vi "MP_Host.vi"() -> ()   [LabVIEW 2019]
uses:
  15fe32d1-7a30-4c0c-a02d-1195f9cfa8e9.vi
  <vilib>/Analysis/baseanly.llb/Mean (DBL).vi
  <vilib>/FPGAPlugInAG/PCIe-7857/niLvFpga_Open_PCIe-7857.vi
  <vilib>/rvi/interface/common/dynamic/niFpgaDynamicAddResources.vi
  <vilib>/FPGAPlugInAG/Dynamic/niLvFpga_Reset_Dynamic.vi
  <vilib>/rvi/interface/common/niFpgaWaitOnOcc.vi
  <vilib>/Utility/error.llb/Error Cluster From Error Code.vi
  <vilib>/FPGAPlugInAG/Dynamic/niLvFpga_Run_Dynamic.vi
  <vilib>/rvi/errors/niLvFpgaAdjustHostInterfaceError.vi
  <vilib>/Utility/file.llb/Write Delimited Spreadsheet (DBL).vi
  <vilib>/FPGAPlugInAG/Dynamic/niLvFpga_Close_Dynamic.vi
  <vilib>/rvi/interface/nirviOpenFPGA/nirviOpenFPGA.xnode
  FPGA Bitfiles/mpembeexp_FPGATarget2_Mpemba1QPDcali_h0D48Adon1s.lvbitx
  Mpemba1_QPDcali.vi
  <vilib>/rvi/interface/nirviMethod/nirviMethod.xnode
  <vilib>/rvi/interface/nirviReadWriteControl/nirviReadWriteControl.xnode
  <vilib>/rvi/interface/nirviCloseFPGA/nirviCloseFPGA.xnode
  <vilib>/rvi/errors/niLvFpgaMergeErrorWithErrorCode.vi
  <vilib>/rvi/interface/Simulation/niFpgaSimulationCallBeginRW.vi
  <vilib>/Analysis/NI_AALBase.lvlib
  NiFpgaLv.dll
  <vilib>/FPGAPlugInAG/Dynamic/niLvFpga_ConfigureFifo_Dynamic.vi
  <vilib>/FPGAPlugInAG/Dynamic/niLvFpga_StartFifo_Dynamic.vi
  <vilib>/FPGAPlugInAG/Dynamic/niLvFpga_ReadFifo_Dynamic.vi
  <vilib>/FPGAPlugInAG/Dynamic/niLvFpga_StopFifo_Dynamic.vi
panel:
  in  "Flat potential\nboundary":dbl=2.0
  out "Drift":waveform(sgl)(graph)
  in  "Reset histogram":bool
  out "Initial position histogram":dynamicdata(graph)
  in  "hw cal time":sgl=50.0
  out "Elements\nremaining":dbl
  in  "AOD_AO4 2":sgl
  in  "AOD_AO0 2":sgl
  in  "Fitting Control":enum32{"Fitting Control", "Fitting Errors"}(tab)
  out "signal offset_X":sgl=5.0
  out "best fit parameters":sgl[](array[numeric])=[0.3806307, 51.013744, 11.326315, -106.03616, 2663.8608, 56396.742]
  in  "initial\nparameters":dbl[](array[numeric])=[0.0, 9.0, 9.5, 0.0, 10.0, 8.0, 0.0]
  in  "Fit?":bool
  in  "Cal px/V":dbl=64.1 format="%#_13g"
  in  "Offset":i32=5
  out "Fitting in \nprogress":bool
  out "residue":dbl
  out "error out":errorcluster
  out "smoothing error":i32
  out "Pos array":sgl[](array[numeric])
  out "Volt":sgl[](array[numeric])
  in  "Use Cal?":bool=TRUE
  in  "V_offset":sgl
  in  "Calibration":T1={"K0"=0.0, "K1"=1.0, "K2"=0.0, "K3"=0.0, "K4"=0.0, "K5"=0.0}
  in  "Bias":sgl
  in  "Fmax":sgl=50.0
  in  "cdfnorm":dbl=1.0 format="%#_16g"
  out "num of protocols":sgl=2126.0
  in  "Calibration ON/OFF":bool=TRUE
  in  "Xoffset":sgl
  in  "Yoffset":sgl
  in  "sum_offset":sgl
  out "Xpot":sgl=-0.1267538 format="%.2f"
  in  "wait time":u8=80
  in  "Temp":i8(ring)=1 items=["Cold", "Warm", "Hot"]
  in  "?":u16(ring) items=["Flat calibration", "Flat cal w drift corr", "No FB", "FB"]
  in  "DW":cluster{"xm":sgl, "Eb":sgl, "Tau":sgl, "dE":sgl}={"xm"=0.5, "Eb"=2.0, "Tau"=70.0, "dE"=1.0} {"dE" format="%#_3g"}
  in  "DL_Y":dbl=2.5 format="%#_13g"
  in  "TL_Y":dbl=2.5 format="%#_13g"
  in  "Stop":bool
  in  "FB time":u32=10
  in  "Triangle wave":T2={"signal offset_X"=5.0, "Scale X"=0.0, "signal offset_Y"=5.0, "Scale Y"=0.0, "Phase Shift"=30}
  in  "Elements":u32=100000
  in  "Data length":dbl=300.0
  out "Done saving":bool
  out "?":dbl=-19.0
  in  "Save Data":bool
  in  "mobX(px/V)":sgl=1.0
  in  "1/Xcali":sgl=1.0
  in  "DX":sgl=53.664
  out "Feedback Loop time":sgl=10.0 format="%.2f"
  out "Underflow":bool
  out "Fx out/Xcorr":sgl=5.0
  out "X":waveform(dbl)(graph)={"t0"=timestamp(0 s since 1904-01-01), "dt"=9.999999747378752e-06, "Y"=array[100000 elements]}
  out "Y":waveform(dbl)(graph)={"t0"=timestamp(0 s since 1904-01-01), "dt"=9.999999747378752e-06, "Y"=array[100000 elements]}
  out "Sum":waveform(dbl)(graph)={"t0"=timestamp(0 s since 1904-01-01), "dt"=9.999999747378752e-06, "Y"=array[100000 elements]}
  in  "Reaverage PS":bool
  out "meanX":dbl=0.10684734082818341 format="%0.5f"
  in  "Xmean":sgl
  out "PSX":dynamicdata(graph)=[{"t0"=timestamp(0 s since 1904-01-01), "dt"=1.0000000252621255, "Y"=array[50000 elements], "attributes"=variant("NI_ChannelName"=variant(string "PSD"))}]
  out "PSY":dynamicdata(graph)=[{"t0"=timestamp(0 s since 1904-01-01), "dt"=1.0000000252621255, "Y"=array[50000 elements], "attributes"=variant("NI_ChannelName"=variant(string "PSD"))}]
  out "PSsum":dynamicdata(graph)=[{"t0"=timestamp(0 s since 1904-01-01), "dt"=1.0000000252621255, "Y"=array[50000 elements], "attributes"=variant("NI_ChannelName"=variant(string "PSD"))}]
  out "Saveloop":u32
  in  "Feedback parameters":T3={"SP_QPDX"=0.0, "alpha"=0.03, "ktrap"=49.2899, "alphacounterX"=0.026}
  in  "TW freq":dbl=1.0
  in  "Normalize signal":bool=TRUE
  out "meanY":dbl=0.08517331748366355 format="%0.5f"
  out "meanZ":dbl=0.8066337188720704 format="%0.4f"
  out "?":errorcluster
  in  "file path (dialog if empty)":path=path "D:/Siddharth/Data/Mpemba replication/2025_04_28/t.txt"
  # "Set both of these to 1"
  # "Set alpha=0.1"
  # "Set cal px/V=60"
  # "Tau=protocol length in us"
  # "Total protocol length = tau+wait time"
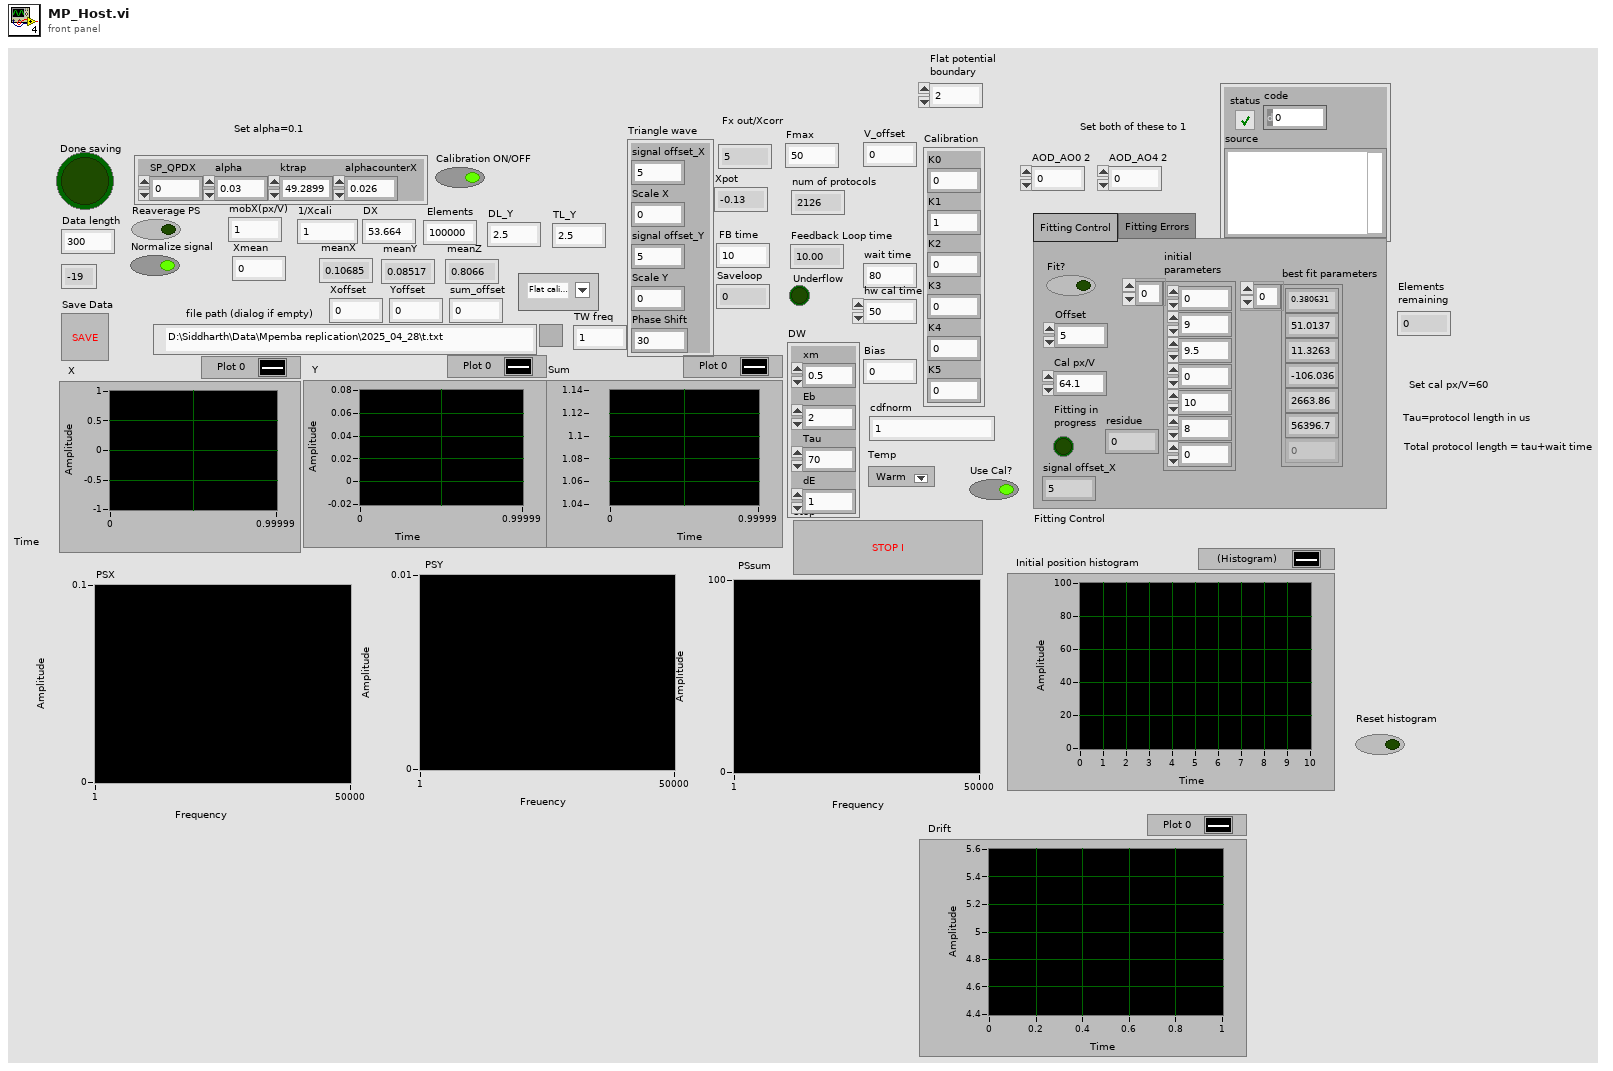
[diagram p1: front panel]
types:
  T1 = cluster{"K0":sgl, "K1":sgl, "K2":sgl, "K3":sgl, "K4":sgl, "K5":sgl}
  T2 = cluster{"signal offset_X":sgl, "Scale X":sgl, "signal offset_Y":sgl, "Scale Y":sgl, "Phase Shift":u32}
  T3 = cluster{"SP_QPDX":sgl, "alpha":sgl, "ktrap":sgl, "alphacounterX":sgl}
  T4 = cluster{"signal offset_X":sgl, dbl, "signal offset_Y":sgl, "Scale Y":sgl, u32}
  T5 = cluster{"[0]":sgl, "[1]":sgl, "[2]":sgl, "[3]":sgl, "[4]":sgl, "[5]":sgl}
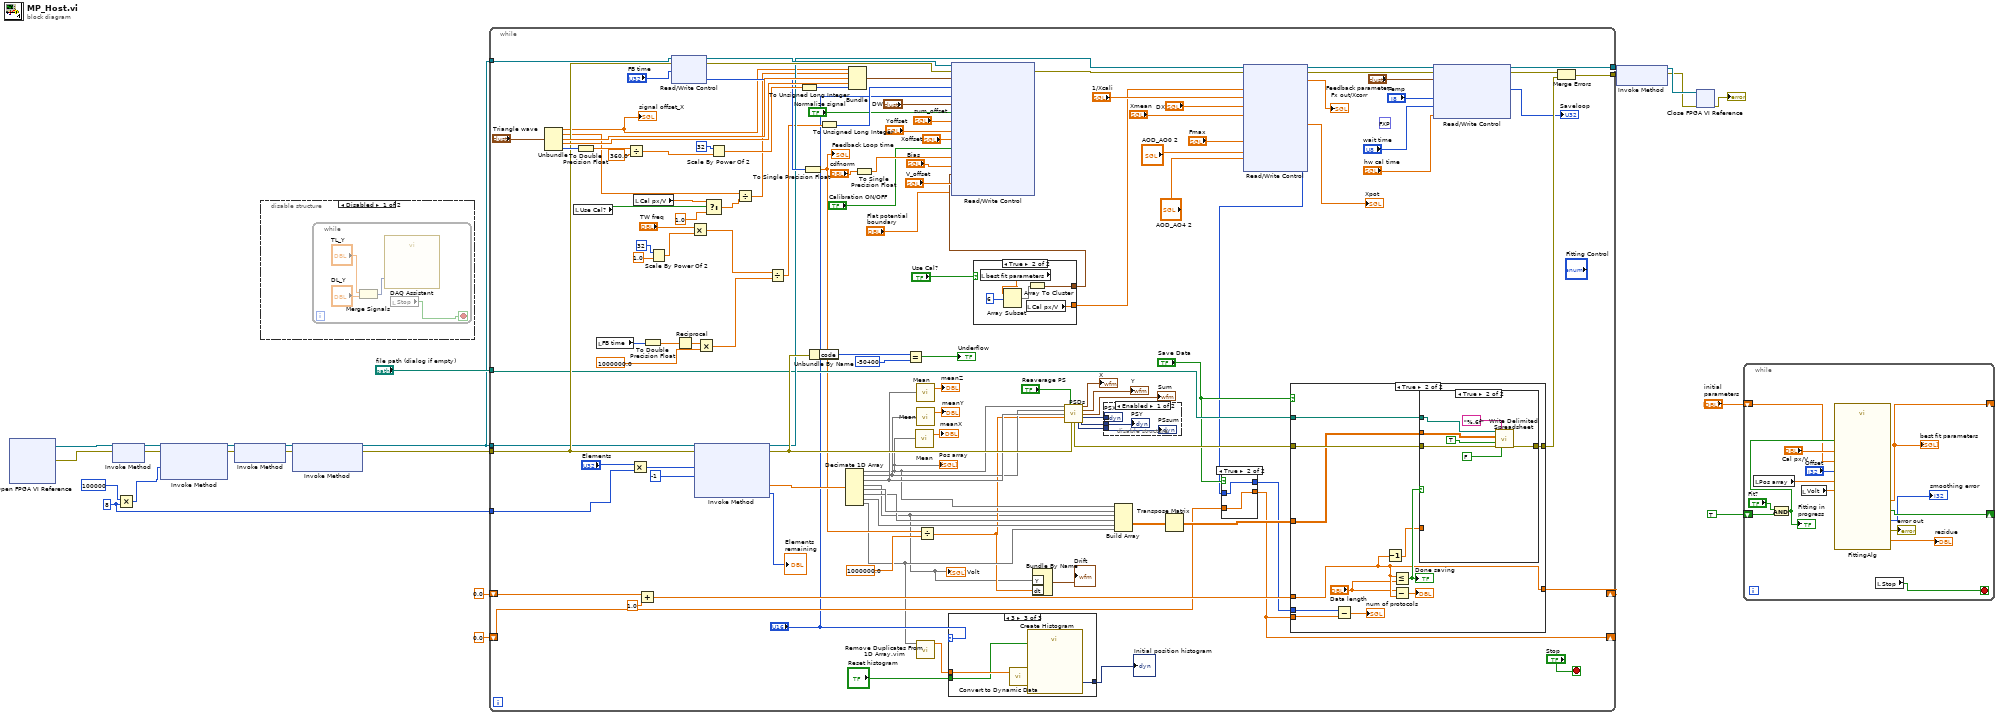
[diagram p0: block diagram]
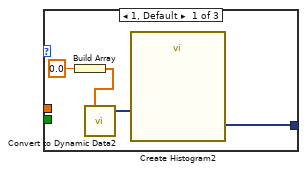
[diagram p3: hidden frame]
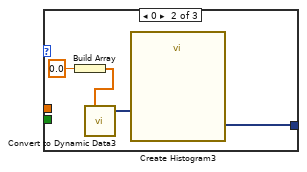
[diagram p4: hidden frame]
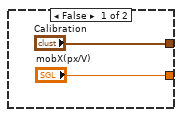
[diagram p5: hidden frame]
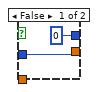
[diagram p6: hidden frame]
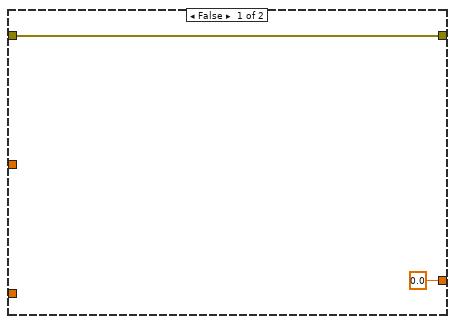
[diagram p8: hidden frame]
diagram:
  w1 = u32 8 ("y")
  n1 = xnode "Open FPGA VI Reference"() -> ("FPGA VI Reference Out"=w7:refnum<k20>, "error out"=w4:errorcluster)  [unwired: 2 in]
  n2 = xnode "Invoke Method"("FPGA VI Reference In"=w7, "error in"=w4) -> ("FPGA VI Reference Out"=w14:refnum<k20>, "error out"=w13:errorcluster)
  n3 = Multiply(x=u32 100000 ("Requested Depth"), y=w1) -> (x*y=w2:u32)
  n4 = xnode "Invoke Method"("FPGA VI Reference In"=w14, "error in"=w13, "Requested Depth"=w2) -> ("FPGA VI Reference Out"=w18:refnum<k20>, "error out"=w17:errorcluster)  [unwired: 1 out]
  n5 = xnode "Invoke Method"("FPGA VI Reference In"=w18, "error in"=w17) -> ("FPGA VI Reference Out"=w20:refnum<k20>, "error out"=w19:errorcluster)
  n6 = disable-structure shown="Disabled" {
    frame Disabled {
      n7 = while {
        stop <- w24 stop-if-true
        n8 = Merge Signals("TL_Y", "DL_Y") -> (w27:dynamicdata)
        n9 = call "DAQ Assistant"("data"=w27) -> ()  [unwired: 17 in, 2 out]
        n10 = local read "Stop"() -> (w24:bool)
      }
    }
    frame Enabled {
    }
  }
  n11 = xnode "Invoke Method"("FPGA VI Reference In"=w20, "error in"=w19) -> ("FPGA VI Reference Out"=w16:refnum<k20>, "error out"=w15:errorcluster)  [unwired: 1 in]
  n12 = while {
    tunnel: w16 -> [w127]
    tunnel: w15 -> [w128]
    tunnel: "file path (dialog if empty)" -> [w96]
    tunnel: [w120] -> w22
    tunnel: [w133] -> w21
    tunnel: w16 -> [w115]
    shift-right: [w124] -> _
    shift-left: 0.0 -> [w123]
    shift-right: [w65] -> _
    shift-left: sgl 0.0 ("num of cycles") -> [w67]
    tunnel: w1 -> [w45]
    stop <- "Stop" stop-if-true
    (unwired) fxp<+,8,7> 50.0 ("Fmax")
    n13 = Unbundle("Triangle wave") -> ("signal offset_X"=w55:sgl, "Scale X"=w33:sgl, "signal offset_Y"=w136:sgl, "Scale Y"=w135:sgl, "Phase Shift"=w137:u32)
    "signal offset_X" <- w55
    n14 = local read "Use Cal?"() -> (w31:bool)
    n15 = To Double Precision Float(number=w137) -> (double precision float=w143:dbl)
    n16 = local read "FB time"() -> (w86:u32)
    n17 = Divide(x=w143, y=360.0) -> (x/y=w141:dbl)
    n18 = Multiply(x="Elements", y=w45) -> (x*y=w129:u32)
    n19 = local read "Cal px/V"() -> (w30:dbl)
    n20 = Add(x=w123, y=1.0) -> (x+y=w125:dbl)
    n21 = To Double Precision Float(number=w86) -> (double precision float=w87:dbl)
    n22 = Scale By Power Of 2(n=i16 32, x=1.0) -> (x*2^n=w91:dbl)
    n23 = xnode "Read/Write Control"("FPGA VI Reference In"=w127, "error in"=w128, "FB Time"="FB time") -> ("FPGA VI Reference Out"=w147:refnum<k20>, "error out"=w116:errorcluster, "FB Time"=w114:u8)
    n24 = Reciprocal(x=w87) -> (1/x=w88:dbl)
    n25 = Multiply(x="TW freq", y=w91) -> (x*y=w84:dbl)
    n26 = xnode "Invoke Method"("FPGA VI Reference In"=w115, "error in"=w128, "Number of Elements"=w129, "Timeout (ms)"=-1) -> ("FPGA VI Reference Out"=w98:refnum<k20>, "error out"=w112:errorcluster, "Data"=w107:sgl[], "Elements Remaining"=→"Elements\nremaining":u32)
    n27 = Multiply(x=w88, y=1000000.0) -> (x*y=w83:dbl)
    n28 = Select(t=w30, s=w31, f=1.0) -> (s? t:f=w29:dbl)
    n29 = Scale By Power Of 2(n=i16 32, x=w141) -> (x*2^n=w139:dbl)
    n30 = Divide(x=w33, y=w29) -> (x/y=w28:dbl)
    n31 = Divide(x=w84, y=w83) -> (x/y=w82:dbl)
    n32 = To Unsigned Long Integer(number=w139) -> (unsigned 32bit integer=w134:u32)
    n33 = To Single Precision Float(number=w114) -> (single precision float=w93:sgl)
    "Feedback Loop time" <- w93
    n34 = Unbundle By Name(w112) -> ("code"=w132:i32)
    n35 = To Unsigned Long Integer(number=w82) -> (unsigned 32bit integer=w81:u32)
    n36 = Decimate 1D Array(w107) -> (w54:sgl[], w72:sgl[], w75:sgl[], w36:sgl[], w76:sgl[], w49:sgl[], w46:sgl[], w42:sgl[])
    "Pos array" <- w54
    "Volt" <- w36
    n37 = Bundle("signal offset_X"=w55, w28, "signal offset_Y"=w136, "Scale Y"=w135, w134) -> (w94:T4)  [unwired: 1 in]
    n38 = To Single Precision Float(number="cdfnorm") -> (single precision float=w59:sgl)
    n39 = Equal?(x=w132, y=-50400) -> (x = y?=→"Underflow":bool)
    n40 = call-poly <vilib>:"Mean.vi"("X"=w54) -> ("mean"=→"meanX":dbl)  [unwired: 1 out]
    n41 = call-poly <vilib>:"Mean.vi"("X"=w75) -> ("mean"=→"meanZ":dbl)  [unwired: 1 out]
    n42 = call "Remove Duplicates From 1D Array.vim"("array"=w42) -> ("array with duplicates removed"=w40:sgl[])  [unwired: 10 in]
    n43 = call-poly <vilib>:"Mean.vi"("X"=w72) -> ("mean"=→"meanY":dbl)  [unwired: 1 out]
    n44 = Divide(x=w93, y=sgl 1000000.0) -> (x/y=w37:sgl)
    n45 = case shown="3" "?" {
      tunnel: [w152 w156 w161] -> w41
      tunnel: w40 -> [_ _ w159]
      tunnel: "Reset histogram" -> [_ _ w158]
      frame 1, Default {
        n46 = Build Array(0.0 ("element")) -> (w150:dbl[])
        n47 = call "Convert to Dynamic Data2"("Array"=w150) -> ("Dynamic Data Type"=w153:dynamicdata)  [unwired: 3 in]
        n48 = call "Create Histogram2"("Signal"=w153) -> ("Histogram"=w152:dynamicdata)  [unwired: 9 in, 1 out]
      }
      frame 0 {
        n49 = Build Array(0.0 ("element")) -> (w154:dbl[])
        n50 = call "Convert to Dynamic Data3"("Array"=w154) -> ("Dynamic Data Type"=w157:dynamicdata)  [unwired: 3 in]
        n51 = call "Create Histogram3"("Signal"=w157) -> ("Histogram"=w156:dynamicdata)  [unwired: 9 in, 1 out]
      }
      frame 3 {
        n52 = call "Convert to Dynamic Data"("Array"=w159) -> ("Dynamic Data Type"=w160:dynamicdata)  [unwired: 3 in]
        n53 = call "Create Histogram"("Reset"=w158, "Signal"=w160) -> ("Histogram"=w161:dynamicdata)  [unwired: 8 in, 1 out]
      }
    }
    "Initial position histogram" <- w41
    n54 = case shown="True" "Use Cal?" {
      tunnel: ["Calibration" w168] -> w58
      tunnel: ["mobX(px/V)" w164] -> w57
      frame False {
      }
      frame True {
        n55 = local read "best fit parameters"() -> (w166:sgl[])
        n56 = Array Subset(array=w166, length=6) -> (w165:sgl[])  [unwired: 1 in]
        n57 = local read "Cal px/V"() -> (w164:dbl)
        n58 = Array To Cluster(array=w165) -> (cluster=w168:T5)
      }
    }
    n59 = xnode "Read/Write Control"("FPGA VI Reference In"=w147, "error in"=w116, "Triangle wave"=w94, "Frequency"=w81, "Enum"="?", "DW"="DW", "Normalize signal"="Normalize signal", "sum_offset"="sum_offset", "Yoffset"="Yoffset", "Xoffset"="Xoffset", "Calibration ON/OFF"="Calibration ON/OFF", "cdfnorm"=w59, "Bias"="Bias", "Calibration"=w58, "V_offset"="V_offset", "Flat potential boundary"="Flat potential\nboundary") -> ("error out"=w97:errorcluster)  [unwired: 1 out]
    n60 = Bundle By Name("Y"=w36, "dt"=w37) -> (→"Drift":waveform(sgl))  [unwired: 1 in]
    n61 = call "PSDs.vi"("X"=w54, "averaging done"="Reaverage PS", "Y"=w72, "sum"=w75, "dt"=w37, "error in (no error)"=w112) -> ("X"=→"X":waveform(dbl), "Y"=→"Y":waveform(dbl), "Sum"=→"Sum":waveform(dbl), "PSDX"=w103:dynamicdata, "error out"=w111:errorcluster, "PSDsum"=w101:dynamicdata, "PSDY"=w102:dynamicdata)  [unwired: 3 in]
    n62 = disable-structure shown="Enabled" {
      disable-tunnel: w103 -> [w175 _]
      disable-tunnel: w102 -> [w174 _]
      disable-tunnel: w101 -> [w173 _]
      frame Enabled {
        "PSX" <- w175
        "PSY" <- w174
        "PSsum" <- w173
      }
      frame Disabled {
      }
    }
    n63 = Build Array(w54, w76, w36, w49, w46, w42) -> (w118:sgl[][])
    n64 = Transpose Matrix(1:w118) -> (0:w146:dbl[][])
    n65 = xnode "Read/Write Control"("FPGA VI Reference In"=w98, "error in"=w97, "MobX(px/V)"=w57, "1/Xcali"="1/Xcali", "DX"="DX", "Xmean"="Xmean", "Fmax"="Fmax", "AOD_AO0 2"="AOD_AO0 2", "AOD_AO4 2"="AOD_AO4 2") -> ("FPGA VI Reference Out"=w122:refnum<k20>, "error out"=w121:errorcluster, "Fx out/Xcorr"=→"Fx out/Xcorr":sgl, "Xpot"=→"Xpot":sgl, "Protocol number"=w47:u32)  [unwired: 1 in]
    n66 = case shown="True" "Save Data" {
      tunnel: [w169 w171] -> w65
      tunnel: w67 -> [_ w171]
      tunnel: [i16 0 ("num of cycles") w172] -> w66
      tunnel: w47 -> [w169 w172]
      frame False {
      }
      frame True {
      }
    }
    n67 = case shown="True" "Save Data" {
      tunnel: w146 -> [_ w184]
      tunnel: w96 -> [_ w189]
      tunnel: w111 -> [w177 w188]
      tunnel: [w177 w187] -> w145
      tunnel: w125 -> [_ w183]
      tunnel: [0.0 w183] -> w124
      tunnel: w66 -> [_ w180]
      tunnel: w65 -> [_ w179]
      frame False {
      }
      frame True {
        n68 = Subtract(x=w180, y=w179) -> (x-y=→"num of protocols":sgl)
        n69 = Decrement(x=w183) -> (x-1=w182:dbl)
        n70 = Less Or Equal?(x=w183, y="Data length") -> (x <= y?=w186:bool)
        "Done saving" <- w186
        n71 = Subtract(x="Data length", y=w183) -> (x-y=→"?":dbl)
        n72 = case shown="True" w186 {
          tunnel: w184 -> [_ w191]
          tunnel: w189 -> [_ w192]
          tunnel: w188 -> [w190 w195]
          tunnel: [w190 w194] -> w187
          tunnel: w182 -> [_ _]
          frame False {
          }
          frame True {
            n73 = call-poly <vilib>:"Write Delimited Spreadsheet.vi"("file path (dialog if empty)"=w192, "format (%.3f)"="%.6f", "2D data"=w191, "append to file? (new file:F)"=TRUE, "error in (no error)"=w195, "transpose? (no:F)"=FALSE) -> ("error out"=w194:errorcluster)  [unwired: 8 in, 1 out]
          }
        }
      }
    }
    n74 = xnode "Read/Write Control"("FPGA VI Reference In"=w122, "error in"=w121, "Feedback parameters"="Feedback parameters", "Temp"="Temp", "wait time"="wait time", "hw cal time"="hw cal time") -> ("FPGA VI Reference Out"=w120:refnum<k20>, "error out"=w119:errorcluster, "Saveloop"=→"Saveloop":u32)
    n75 = Merge Errors(w119, w145) -> (w133:errorcluster)
  }
  n76 = xnode "Invoke Method"("FPGA VI Reference In"=w22, "error in"=w21) -> ("FPGA VI Reference Out"=w12:refnum<k20>, "error out"=w11:errorcluster)
  n77 = xnode "Close FPGA VI Reference"("FPGA VI Reference In"=w12, "error in"=w11) -> ("error out"=→"?":errorcluster)
  n78 = while {
    shift-right: [w211] -> _
    shift-left: "initial\nparameters" -> [w199]
    shift-right: [w203] -> _
    shift-left: TRUE -> [w206]
    stop <- w198 stop-if-true
    n79 = local read "Pos array"() -> (w210:sgl[])
    n80 = And(x="Fit?", y=w206) -> (x .and. y?=w204:bool)
    "Fitting in \nprogress" <- w204
    n81 = local read "Volt"() -> (w209:sgl[])
    n82 = call "FittingAlg.vi"("Pos"=w210, "Cal px/V"="Cal px/V", "initial parameters"=w199, "Volt"=w209, "Boolean in"=w204, "Offset"="Offset") -> ("error"=→"smoothing error":i32, "best fit parameters"=w211:dbl[], "Boolean out"=w203:bool, "residue"=→"residue":dbl, "error out"=→"error out":errorcluster)  [unwired: 5 in]
    "best fit parameters" <- w211
    n83 = local read "Stop"() -> (w198:bool)
  }
